vi "A170316-11-Main-large.vi"() -> ()   [LabVIEW 2020]
uses:
  System.Windows.Forms
  Database/Global1.vi
  Global_Variable/Global.vi
  <userlib>/_MGI/Menu Building/MenuTypes/MenuStrip/MGI_MenuStrip.lvclass
  <userlib>/_MGI/Menu Building/MenuItemStatusChange/MGI_MenuItemStatusChange.lvclass
  Global_Variable/A170316-11.vi
  Libraries/S7/S7.lvlib
panel:
  out "PLC":bool
  in  "模式切换":refnum<vi>
  out "管柱码":string
  out "电机自动":bool
  out "上序状态":string
  out "ECU前序显示字":string
  out "电机前序显示字":string
  out "ECU装配\n前序状态":bool
  out "上序状态":bool
  out "电机码":string
  out "电机工位管柱码":string
  out "控制器码":string
  out "ECU自动":bool
  out "电机安装数量":u32
  out "ECU结果显示":string
  out "电机结果显示":string
  in  "质量报警":bool caption="布尔"
  in  "设备缺料":bool caption="布尔"
  in  "设备故障":bool caption="布尔"
  in  "设备离线":bool caption="布尔"
  in  "设备正常":bool caption="布尔"
  in  "菜单":refnum<k24>(container)
  out "检测结果":bool
  in  "批次信息":string[][](table)
  out "提示信息":string
  out "错误":bool
  out "时间字符串":string
  out "日期字符串":string
  out "userStatus":string caption="用户状态"
  out "userName":string caption="用户名"
  out "安装支架数量":u32
  out "ECU工位管柱码":string
  out "connectionMode":string caption="联机类型"
  out "产品型号":string
  in  "更换产品":refnum<vi>
  # "调节机构装配"
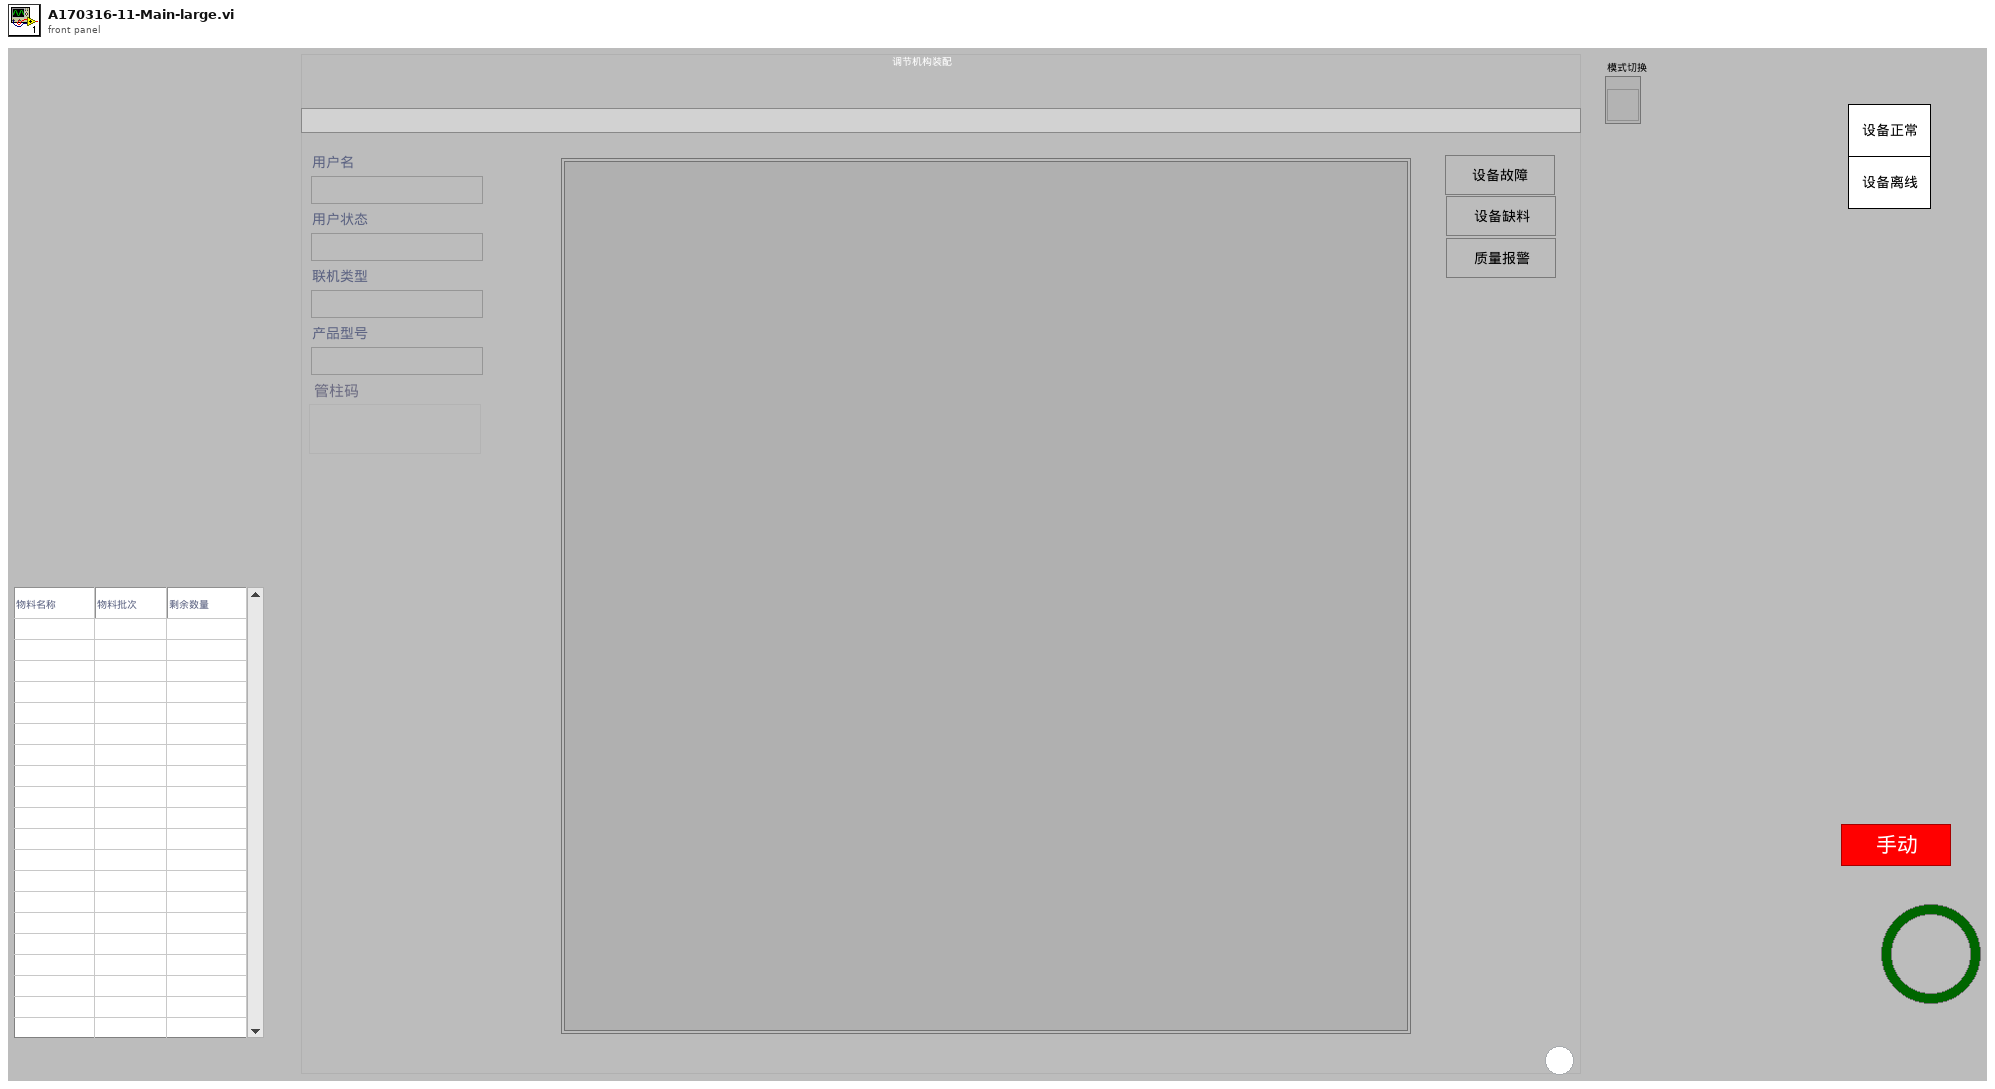
[diagram p1: front panel]
types:
  T1 = typedef "S7.lvlib/Broadcast Events--cluster.ctl" = cluster{"Module Did Init":refnum<user-event>, "Status Updated":refnum<user-event>, "Error Reported":refnum<user-event>, "Module Did Stop":refnum<user-event>, "Update Module Execution Status":refnum<user-event>}
  T2 = enum32{"Invalid", "Standard", "Closed", "Hidden", "Minimized", "Maximized"}
  T3 = enum32{"invalid app kind", "Development System", "Run Time System", "Student Edition", "Embedded LabVIEW", "Evaluation", "Custom"}
  T4 = cluster{"Core":cluster{"Current VI Reference":refnum<vi>, "Close Panel on Exit?":bool}, "Your Boolean data":bool, "Your string data":string}
  T5 = cluster{"Current VI Reference":refnum<vi>, "Close Panel on Exit?":bool}
  T6 = cluster{"用户编号":string, "用户名":string, "用户密码(密文)":string, "用户权限":string}
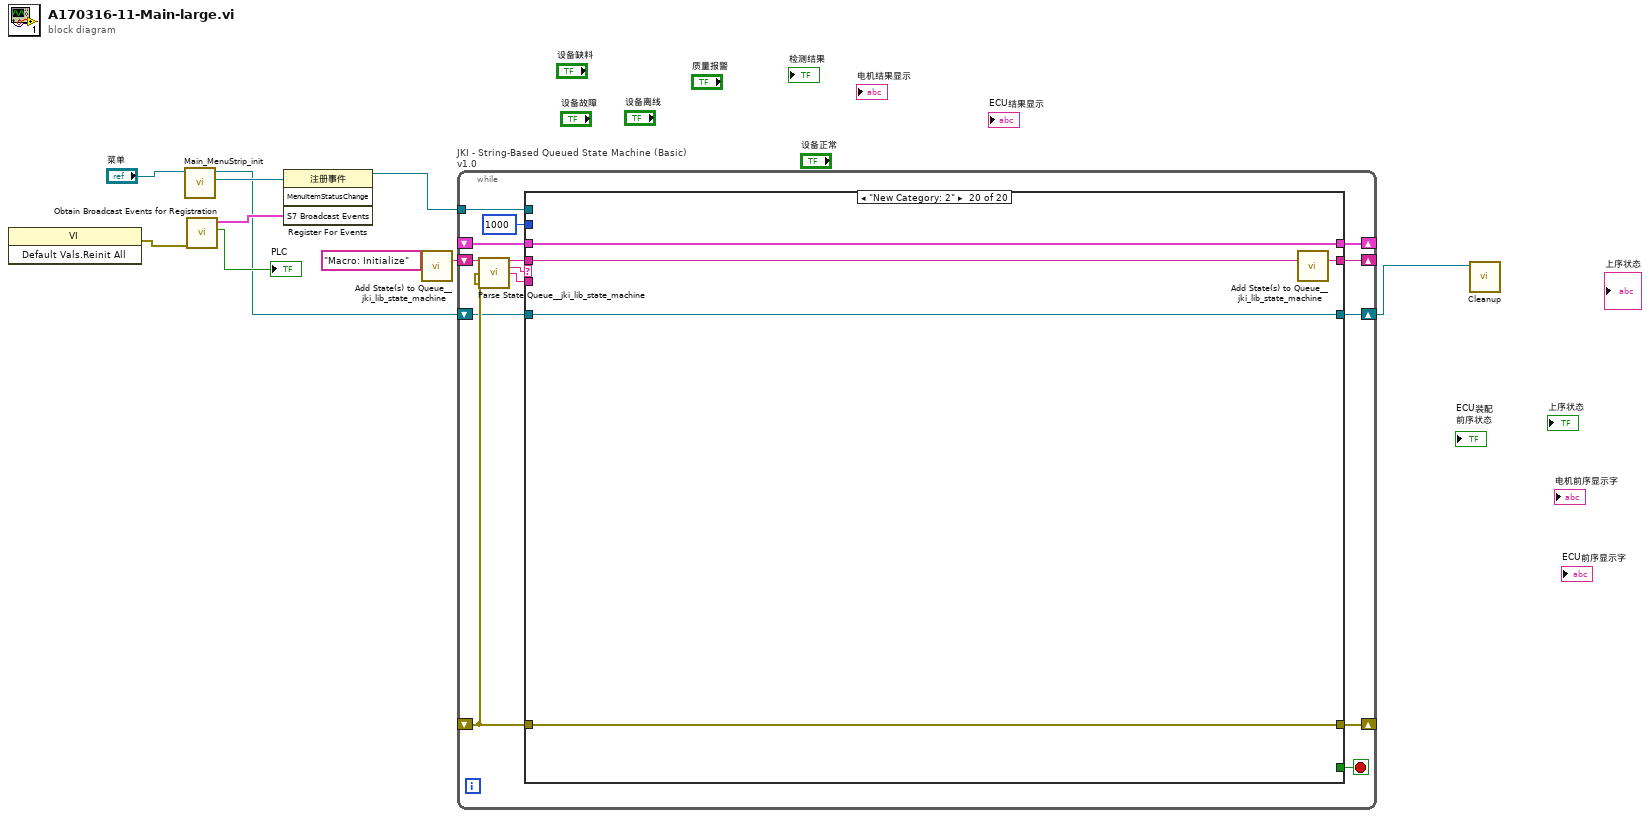
[diagram p0: block diagram]
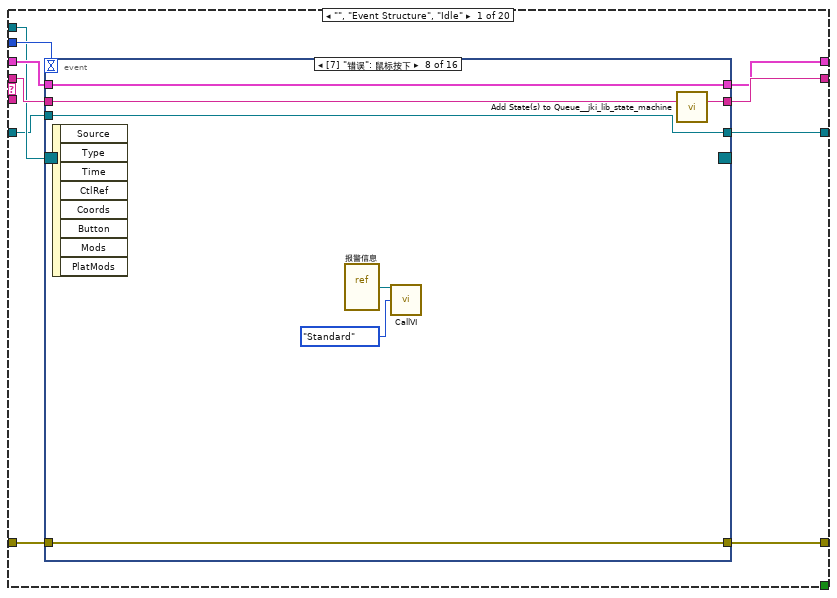
[diagram p2: hidden frame]
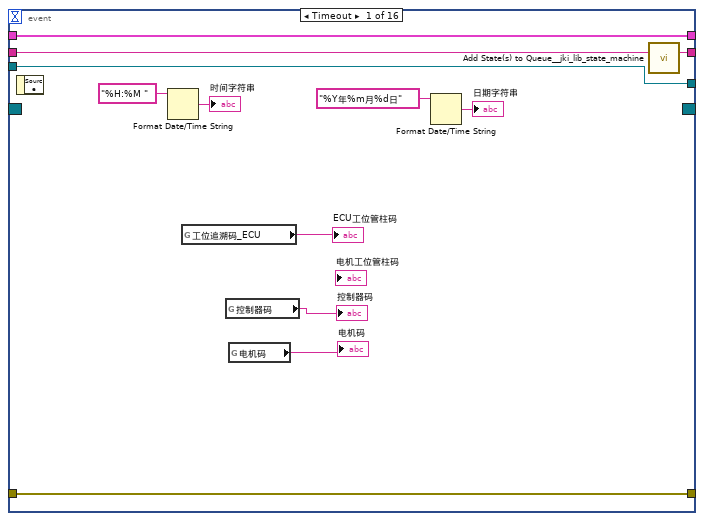
[diagram p3: hidden frame]
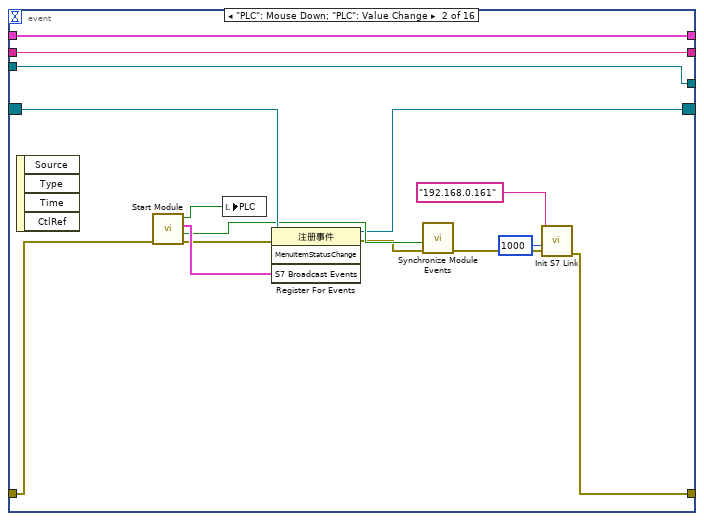
[diagram p4: hidden frame]
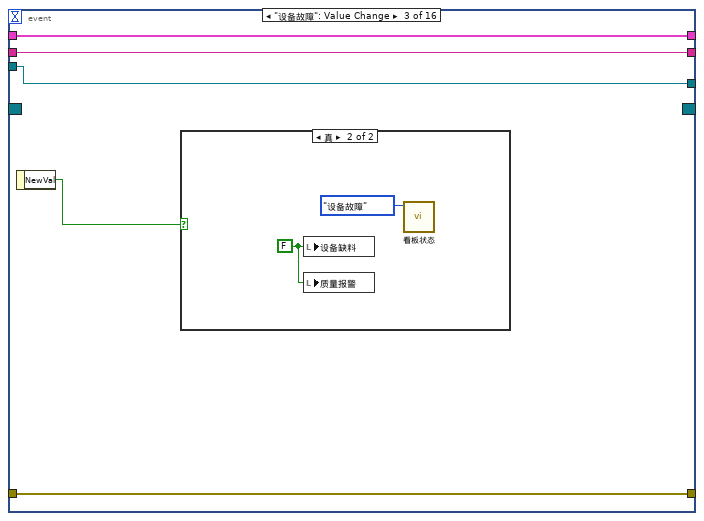
[diagram p5: hidden frame]
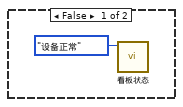
[diagram p6: hidden frame]
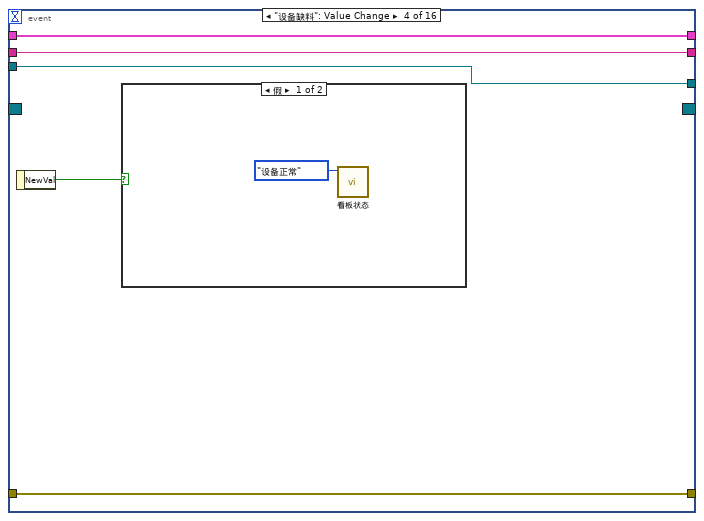
[diagram p7: hidden frame]
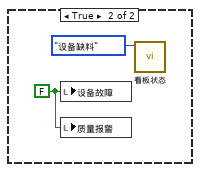
[diagram p8: hidden frame]
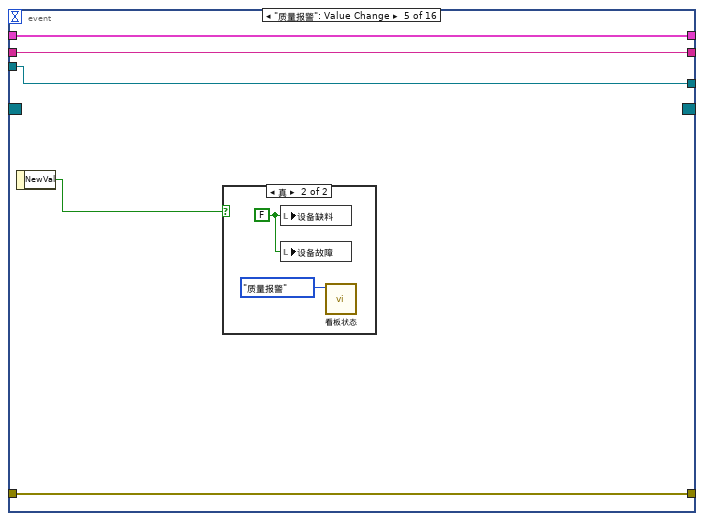
[diagram p9: hidden frame]
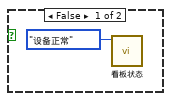
[diagram p10: hidden frame]
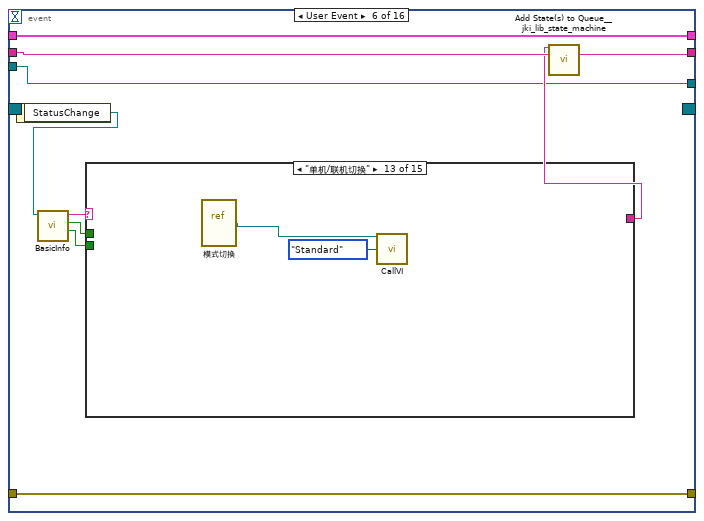
[diagram p11: hidden frame]
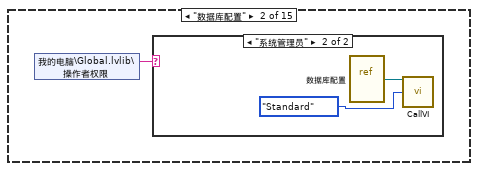
[diagram p13: hidden frame]
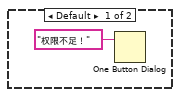
[diagram p14: hidden frame]
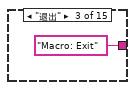
[diagram p15: hidden frame]
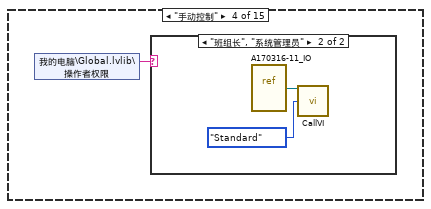
[diagram p16: hidden frame]
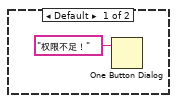
[diagram p17: hidden frame]
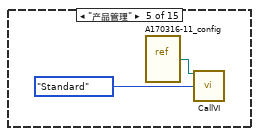
[diagram p18: hidden frame]
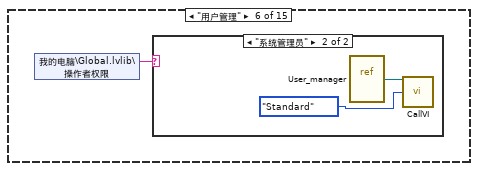
[diagram p19: hidden frame]
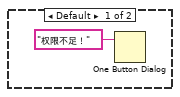
[diagram p20: hidden frame]
diagram:
  n1 = invoke class="VI" method="Default Vals.Reinit All"() -> (error out=w3:errorcluster)  [unwired: 3 in, 2 out]
  n2 = call "Main_MenuStrip_init.vi"("MenuStrip"="菜单") -> ("MenuItemStatusChange"=w6:refnum<user-event>, "Menu out"=w2:refnum<class "MGI_MenuStrip.lvclass">)  [unwired: 9 in]
  n3 = call "Obtain Broadcast Events for Registration.vi"("error in (no error)"=w3) -> ("Already running?"=→"PLC":bool, "S7 Broadcast Events"=w5:T1)  [unwired: 8 in, 1 out]
  n4 = register-events(w6, w5) -> (reference out=w7:refnum<event-registration>)  [unwired: 2 in, 1 out]
  n5 = call <vilib>:"Add State(s) to Queue__jki_lib_state_machine.vi"("State(s) in (\"\")"="Macro: Initialize") -> ("States Out"=w10:string)  [unwired: 14 in]
  n6 = while "JKI - String-Based Queued State Machine (Basic) v1.0" {
    shift-right: [w17] -> _
    shift-left: _ -> [w16]
    shift-right: [w20] -> _
    shift-left: _ -> [w14]
    shift-right: [w19] -> _
    shift-left: w10 -> [w21]
    tunnel: w7 -> [w13]
    shift-right: [w11] -> w1
    shift-left: w2 -> [w12]
    stop <- w18 stop-if-true
    n7 = call <vilib>:"Parse State Queue__jki_lib_state_machine.vi"("State Queue"=w21, "Error In (no error)"=w14) -> ("Remaining States"=w23:string, "Current State"=w24:string, "Arguments"=w22:string)  [unwired: 11 in]
    n8 = case shown="\"New Category: 2\"" w24 {
      selector: w24 -> [_ _ w268 _ _ _ _ _ _ _ _ _ _ _ _ _ _ _ _ _]
      tunnel: w23 -> [w34 w266 w272 w291 w298 w304 w309 w317 w324 w329 w342 w347 w407 w419 w446 w452 w468 w473 w478 w483]
      tunnel: w22 -> [_ _ _ _ _ _ _ _ _ _ _ _ w402 w413 _ _ _ _ _ _]
      tunnel: w16 -> [w32 w263 w270 w282 w295 w302 w306 _ w319 w326 w340 w345 w405 w415 w443 w449 w465 w470 w475 w480]
      tunnel: [w31 w264 w274 w288 errorcluster {"status"=FALSE, "code"=0, "source"=""} ("error out") w301 w307 w314 w320 w327 w339 w344 w403 w416 w444 w450 w466 w471 w476 w481] -> w20
      tunnel: w14 -> [w30 w264 w273 w288 w294 w301 w307 w314 w321 w327 w338 w344 w404 w417 w444 w450 w466 w471 w476 w481]
      tunnel: [w33 w265 w271 w290 w297 w303 w308 w316 w323 w328 w341 w346 w406 w418 w445 w451 w467 w472 w477 w482] -> w19
      tunnel: [_ _ _ _ _ TRUE _ _ _ _ _ _ _ _ _ _ _ _ _ _] -> w18
      tunnel: [w29 w263 w270 w289 w295 w302 w306 w315 w319 w326 w340 w345 w405 w415 w443 w449 w465 w470 w475 w480] -> w17
      tunnel: 1000 ("Timeout") -> [w28 _ _ _ _ _ _ _ _ _ _ _ _ _ _ _ _ _ _ _]
      tunnel: w13 -> [w27 _ _ _ _ _ _ _ _ _ _ _ _ _ _ _ _ _ _ _]
      tunnel: w12 -> [w26 w262 w267 w279 w292 w299 w305 w310 w318 w325 w330 w343 w401 w412 w442 w447 w453 w469 w474 w479]
      tunnel: [w25 w262 w267 w279 w292 w299 w305 w310 w318 w325 w330 w343 w401 w412 w442 w447 w453 w469 w474 w479] -> w11
      frame "", "Event Structure", "Idle" {
        n9 = event shown="[7] \"错误\": 鼠标按下" {
          selector: w27 -> [_ w59 _ _ _ _ _ _ _ _ _ _ _ _ _ _]
          dyn-events: [_ w50 _ _ _ _ _ _ _ _ _ _ _ _ _ _] -> _
          timeout: w28 -> [_ _ _ _ _ _ _ _ _ _ _ _ _ _ _ _]
          tunnel: w34 -> [w46 w48 w65 w73 w81 w90 w143 w194 w201 w225 w229 w234 w239 w246 w255 w258]
          tunnel: [w45 w48 w65 w73 w81 w89 w141 w195 w201 w225 w229 w234 w239 w244 w254 w259] -> w33
          tunnel: w32 -> [w43 w49 w66 w74 w82 w91 w142 w196 w202 w226 w228 w235 w240 w245 w252 w261]
          tunnel: [w44 w51 w64 w72 w80 w87 w144 w193 w200 w224 w227 w232 w237 w242 w253 w260] -> w31
          tunnel: w30 -> [w44 w61 w64 w72 w80 w87 w144 w193 w200 w224 w227 w232 w237 w242 w253 w260]
          tunnel: [w43 w49 w66 w74 w82 w91 w142 w196 w202 w226 w228 w235 w240 w245 w252 w261] -> w29
          tunnel: w26 -> [w35 w47 w62 w70 w78 w86 w140 w190 w197 w223 w230 w233 w238 w243 _ _]
          tunnel: [w35 w47 w62 w70 w78 w86 w140 w190 w197 w223 w230 w233 w238 w243 _ _] -> w25
          event Timeout {
            n10 = event-data() -> ()  [unwired: 1 in, 1 out]
            n11 = Format Date/Time String(time format string (%c)="%H:%M ") -> (date/time string=→"时间字符串":string)  [unwired: 2 in]
            n12 = global read "Global1.vi" "工位追溯码_ECU"() -> (→"ECU工位管柱码":string)
            n13 = global read "Global1.vi" "控制器码"() -> (→"控制器码":string)
            n14 = global read "Global1.vi" "电机码"() -> (→"电机码":string)
            n15 = Format Date/Time String(time format string (%c)="%Y年%m月%d日") -> (date/time string=→"日期字符串":string)  [unwired: 2 in]
            n16 = call <vilib>:"Add State(s) to Queue__jki_lib_state_machine.vi"("State(s) in (\"\")"=w46) -> ("States Out"=w45:string)  [unwired: 14 in]
          }
          event "PLC": Mouse Down; "PLC": Value Change {
            n17 = event-data() -> ()  [unwired: 1 in, 4 out]
            n18 = call "Start Module.vi"("error in (no error)"=w61) -> ("error out"=w57:errorcluster, "Wait for Event Sync?"=w56:bool, "S7 Broadcast Events"=w58:T1, "Module Was Already Running?"=w60:bool)  [unwired: 7 in]
            n19 = local write "PLC"(w60) -> ()
            n20 = register-events(reference=w59, error in=w57, w58) -> (reference out=w50:refnum<event-registration>, error out=w55:errorcluster)  [unwired: 1 in]
            n21 = call "Synchronize Module Events.vi"("error in (no error)"=w55, "Wait for Event Sync?"=w56) -> ("error out"=w54:errorcluster)  [unwired: 9 in]
            n22 = call "Init S7 Link.vi"("error in (no error)"=w54, "超时"=1000, "IP"="192.168.0.161") -> ("error out"=w51:errorcluster)  [unwired: 8 in]
          }
          event "设备故障": Value Change {
            n23 = event-data() -> ("NewVal"=w63:bool)  [unwired: 1 in]
            n24 = case shown="真" w63 {
              frame False {
                n25 = call "看板状态.vi"("设备状态"=enum16{"设备离线", "设备正常", "设备缺料", "设备故障", "质量报警"}."设备正常") -> ()  [unwired: 10 in, 1 out]
              }
              frame True {
                w68 = FALSE ("质量报警")
                n26 = local write "设备缺料"(w68) -> ()
                n27 = local write "质量报警"(w68) -> ()
                n28 = call "看板状态.vi"("设备状态"=enum16{"设备离线", "设备正常", "设备缺料", "设备故障", "质量报警"}."设备故障") -> ()  [unwired: 10 in, 1 out]
              }
            }
          }
          event "设备缺料": Value Change {
            n29 = event-data() -> ("NewVal"=w71:bool)  [unwired: 1 in]
            n30 = case shown="假" w71 {
              frame False {
                n31 = call "看板状态.vi"("设备状态"=enum16{"设备离线", "设备正常", "设备缺料", "设备故障", "质量报警"}."设备正常") -> ()  [unwired: 10 in, 1 out]
              }
              frame True {
                w76 = FALSE ("质量报警")
                n32 = local write "设备故障"(w76) -> ()
                n33 = local write "质量报警"(w76) -> ()
                n34 = call "看板状态.vi"("设备状态"=enum16{"设备离线", "设备正常", "设备缺料", "设备故障", "质量报警"}."设备缺料") -> ()  [unwired: 10 in, 1 out]
              }
            }
          }
          event "质量报警": Value Change {
            n35 = event-data() -> ("NewVal"=w79:bool)  [unwired: 1 in]
            n36 = case shown="真" w79 {
              frame False {
                n37 = call "看板状态.vi"("设备状态"=enum16{"设备离线", "设备正常", "设备缺料", "设备故障", "质量报警"}."设备正常") -> ()  [unwired: 10 in, 1 out]
              }
              frame True {
                w84 = FALSE ("质量报警")
                n38 = local write "设备缺料"(w84) -> ()
                n39 = local write "设备故障"(w84) -> ()
                n40 = call "看板状态.vi"("设备状态"=enum16{"设备离线", "设备正常", "设备缺料", "设备故障", "质量报警"}."质量报警") -> ()  [unwired: 10 in, 1 out]
              }
            }
          }
          event User Event {
            n41 = event-data() -> ("StatusChange"=w92:refnum<class "MGI_MenuItemStatusChange.lvclass">)  [unwired: 1 in]
            n42 = call <userlib>:"BasicInfo.vi"("MGI_MenuItemStatusChange in"=w92) -> ("Enabled?"=w95:bool, "Checked?"=w94:bool, "Tag"=w93:string)  [unwired: 7 in, 1 out]
            n43 = case shown="\"单机/联机切换\"" w93 {
              tunnel: w94 -> [_ _ _ _ _ _ _ _ _ _ _ _ _ _ _]
              tunnel: w95 -> [_ _ _ _ _ _ _ _ _ _ _ _ _ _ _]
              tunnel: [_ _ "Macro: Exit" _ _ _ _ _ _ _ _ _ _ _ _] -> w88
              frame Default {
              }
              frame "数据库配置" {
                n44 = shared-variable "我的电脑\\Global.lvlib\\操作者权限"() -> (w96:string)  [unwired: 1 in, 1 out]
                n45 = case shown="\"系统管理员\"" w96 {
                  frame Default {
                    n46 = One Button Dialog(message="权限不足！" ("消息")) -> ()  [unwired: 1 in, 1 out]
                  }
                  frame "系统管理员" {
                    n47 = vi-ref "数据库配置.vi"() -> (w99:refnum<vi>)
                    n48 = call "CallVI.vi"("VI引用"=w99, "状态"=T2."Standard") -> ()  [unwired: 11 in, 3 out]
                  }
                }
              }
              frame "退出" {
              }
              frame "手动控制" {
                n49 = shared-variable "我的电脑\\Global.lvlib\\操作者权限"() -> (w101:string)  [unwired: 1 in, 1 out]
                n50 = case shown="\"班组长\", \"系统管理员\"" w101 {
                  frame Default {
                    n51 = One Button Dialog(message="权限不足！" ("消息")) -> ()  [unwired: 1 in, 1 out]
                  }
                  frame "班组长", "系统管理员" {
                    n52 = vi-ref "A170316-11_IO.vi"() -> (w104:refnum<vi>)
                    n53 = call "CallVI.vi"("VI引用"=w104, "状态"=T2."Standard") -> ()  [unwired: 11 in, 3 out]
                  }
                }
              }
              frame "产品管理" {
                n54 = vi-ref "A170316-11_config.vi"() -> (w106:refnum<vi>)
                n55 = call "CallVI.vi"("VI引用"=w106, "状态"=T2."Standard") -> ()  [unwired: 11 in, 3 out]
              }
              frame "用户管理" {
                n56 = shared-variable "我的电脑\\Global.lvlib\\操作者权限"() -> (w107:string)  [unwired: 1 in, 1 out]
                n57 = case shown="\"系统管理员\"" w107 {
                  frame Default {
                    n58 = One Button Dialog(message="权限不足！" ("消息")) -> ()  [unwired: 1 in, 1 out]
                  }
                  frame "系统管理员" {
                    n59 = vi-ref "User_manager.vi"() -> (w110:refnum<vi>)
                    n60 = call "CallVI.vi"("VI引用"=w110, "状态"=T2."Standard") -> ()  [unwired: 11 in, 3 out]
                  }
                }
              }
              frame "编码规则" {
                n61 = shared-variable "我的电脑\\Global.lvlib\\操作者权限"() -> (w111:string)  [unwired: 1 in, 1 out]
                n62 = case shown="\"班组长\", \"工艺管理员\", \"系统管理员\"" w111 {
                  frame Default {
                    n63 = One Button Dialog(message="权限不足！" ("消息")) -> ()  [unwired: 1 in, 1 out]
                  }
                  frame "班组长", "工艺管理员", "系统管理员" {
                    n64 = vi-ref "编码规则设置.vi"() -> (w114:refnum<vi>)
                    n65 = call "CallVI.vi"("VI引用"=w114, "状态"=T2."Standard") -> ()  [unwired: 11 in, 3 out]
                  }
                }
              }
              frame "易损件管理" {
                n66 = vi-ref "易损件管理.vi"() -> (w116:refnum<vi>)
                n67 = call "CallVI.vi"("VI引用"=w116, "状态"=T2."Standard") -> ()  [unwired: 11 in, 3 out]
              }
              frame "物料批次管理" {
                n68 = vi-ref "批次管理.vi"() -> (w118:refnum<vi>)
                n69 = call "CallVI.vi"("VI引用"=w118, "状态"=T2."Standard") -> ()  [unwired: 11 in, 3 out]
              }
              frame "设备管理" {
                n70 = vi-ref "注册设备.vi"() -> (w120:refnum<vi>)
                n71 = call "CallVI.vi"("VI引用"=w120, "状态"=T2."Standard") -> ()  [unwired: 11 in, 3 out]
              }
              frame "报表" {
                n72 = call "文件对话框2"("start path"=path "D:/report", "prompt"="打开报表", "pattern (all files)"="*.doc;*.docx", "pattern label"="Word 文档") -> ("selected path"=w121:path, "error out"=w122:errorcluster)  [unwired: 8 in, 2 out]
                n73 = case shown="无错误" w122 {
                  selector: w122 -> [w128 w130]
                  tunnel: w121 -> [w129 _]
                  frame No Error {
                    w127 = 1 items=["Normal", "Maximize", "Minimize"] ("cpubbs_WindowState")
                    n74 = call "Open_Word.vi"("File Path"=w129, "cpubbs_WindowState"=w127, "错误输入（无错误）"=w128) -> ()  [unwired: 12 in, 1 out]
                  }
                  frame Error {
                    n75 = call <vilib>:"Clear Errors.vi"("error in (no error)"=w130) -> ()  [unwired: 5 in, 2 out]
                  }
                }
              }
              frame "报警信息" {
                n76 = vi-ref "报警信息.vi"() -> (w132:refnum<vi>)
                n77 = call "CallVI.vi"("VI引用"=w132, "状态"=T2."Standard") -> ()  [unwired: 11 in, 3 out]
              }
              frame "单机/联机切换" {
                n78 = vi-ref "模式切换.vi"() -> (w133:refnum<vi>)
                n79 = call "CallVI.vi"("VI引用"=w133, "状态"=T2."Standard") -> ()  [unwired: 11 in, 3 out]
              }
              frame "关于" {
                n80 = vi-ref "About.vi"() -> (w136:refnum<vi>)
                n81 = call "CallVI.vi"("VI引用"=w136, "状态"=T2."Standard") -> ()  [unwired: 11 in, 3 out]
              }
              frame "操作演示" {
                n82 = call <vilib>:"Application Directory.vi"() -> ("Application Directory"=w139:path)
                n83 = Build Path(base path=w139, name or relative path="操作演示" ("名称或相对路径")) -> (appended path=w138:path)
                n84 = call "自动播放ppt.vi"("路径"=w138) -> ()  [unwired: 10 in, 1 out]
              }
            }
            n85 = call <vilib>:"Add State(s) to Queue__jki_lib_state_machine.vi"("State(s) in Front (\"\")"=w88, "State(s) in (\"\")"=w90) -> ("States Out"=w89:string)  [unwired: 13 in]
          }
          event Menu Selection (User) {
            n86 = event-data() -> ("ItemTag"=w145:string)  [unwired: 1 in, 6 out]
            n87 = case shown="\"易损件管理\"" w145 {
              frame "假", Default {
              }
              frame "数据库配置" {
                n88 = shared-variable "我的电脑\\Global.lvlib\\操作者权限"() -> (w146:string)  [unwired: 1 in, 1 out]
                n89 = case shown="\"系统管理员\"" w146 {
                  frame Default {
                    n90 = One Button Dialog(message="权限不足！" ("消息")) -> ()  [unwired: 1 in, 1 out]
                  }
                  frame "系统管理员" {
                    n91 = vi-ref "数据库配置.vi"() -> (w149:refnum<vi>)
                    n92 = call "CallVI.vi"("VI引用"=w149, "状态"=T2."Standard") -> ()  [unwired: 11 in, 3 out]
                  }
                }
              }
              frame "退出" {
                n93 = Quit LabVIEW() -> ()  [unwired: 1 in]
              }
              frame "手动控制" {
                n94 = shared-variable "我的电脑\\Global.lvlib\\操作者权限"() -> (w150:string)  [unwired: 1 in, 1 out]
                n95 = case shown="\"班组长\", \"系统管理员\"" w150 {
                  frame Default {
                    n96 = One Button Dialog(message="权限不足！" ("消息")) -> ()  [unwired: 1 in, 1 out]
                  }
                  frame "班组长", "系统管理员" {
                    n97 = vi-ref "A170316-11_IO.vi"() -> (w153:refnum<vi>)
                    n98 = call "CallVI.vi"("VI引用"=w153, "状态"=T2."Standard") -> ()  [unwired: 11 in, 3 out]
                  }
                }
              }
              frame "半自动控制" {
                n99 = disable-structure shown="启用" {
                  frame Disabled {
                    n100 = shared-variable "我的电脑\\Global.lvlib\\操作者权限"() -> (w154:string)  [unwired: 1 in, 1 out]
                    n101 = case shown="\"班组长\", \"系统管理员\"" w154 {
                      frame Default {
                        n102 = One Button Dialog(message="权限不足！" ("消息")) -> ()  [unwired: 1 in, 1 out]
                      }
                      frame "班组长", "系统管理员" {
                        n103 = call "CallVI.vi"("VI引用"=refnum<vi> refnum, "状态"=T2."Maximized") -> ()  [unwired: 11 in, 3 out]
                      }
                    }
                  }
                  frame Enabled {
                    n104 = One Button Dialog(message="当前设备不具备半自动功能！" ("消息")) -> ()  [unwired: 1 in, 1 out]
                  }
                }
              }
              frame "产品管理" {
                n105 = vi-ref "A170316-11_config.vi"() -> (w160:refnum<vi>)
                n106 = call "CallVI.vi"("VI引用"=w160, "状态"=T2."Standard") -> ()  [unwired: 11 in, 3 out]
              }
              frame "系统配置" {
              }
              frame "用户管理" {
                n107 = shared-variable "我的电脑\\Global.lvlib\\操作者权限"() -> (w161:string)  [unwired: 1 in, 1 out]
                n108 = case shown="\"系统管理员\"" w161 {
                  frame Default {
                    n109 = One Button Dialog(message="权限不足！" ("消息")) -> ()  [unwired: 1 in, 1 out]
                  }
                  frame "系统管理员" {
                    n110 = vi-ref "User_manager.vi"() -> (w164:refnum<vi>)
                    n111 = call "CallVI.vi"("VI引用"=w164, "状态"=T2."Standard") -> ()  [unwired: 11 in, 3 out]
                  }
                }
              }
              frame "编码规则" {
                n112 = shared-variable "我的电脑\\Global.lvlib\\操作者权限"() -> (w165:string)  [unwired: 1 in, 1 out]
                n113 = case shown="\"班组长\", \"工艺管理员\", \"系统管理员\"" w165 {
                  frame Default {
                    n114 = One Button Dialog(message="权限不足！" ("消息")) -> ()  [unwired: 1 in, 1 out]
                  }
                  frame "班组长", "工艺管理员", "系统管理员" {
                    n115 = vi-ref "编码规则设置.vi"() -> (w168:refnum<vi>)
                    n116 = call "CallVI.vi"("VI引用"=w168, "状态"=T2."Standard") -> ()  [unwired: 11 in, 3 out]
                  }
                }
              }
              frame "易损件管理" {
                n117 = vi-ref "易损件管理.vi"() -> (w170:refnum<vi>)
                n118 = call "CallVI.vi"("VI引用"=w170, "状态"=T2."Standard") -> ()  [unwired: 11 in, 3 out]
              }
              frame "物料批次管理" {
                n119 = vi-ref "批次管理.vi"() -> (w172:refnum<vi>)
                n120 = call "CallVI.vi"("VI引用"=w172, "状态"=T2."Standard") -> ()  [unwired: 11 in, 3 out]
              }
              frame "打开报表" {
                n121 = call "文件对话框"("start path"=path "D:/report", "prompt"="打开报表", "pattern (all files)"="*.doc;*.docx", "pattern label"="Word 文档") -> ("selected path"=w173:path, "error out"=w174:errorcluster)  [unwired: 8 in, 2 out]
                n122 = case shown="无错误" w174 {
                  selector: w174 -> [w180 w182]
                  tunnel: w173 -> [w181 _]
                  frame No Error {
                    w179 = 1 items=["Normal", "Maximize", "Minimize"] ("cpubbs_WindowState")
                    n123 = call "Open_Word.vi"("File Path"=w181, "cpubbs_WindowState"=w179, "错误输入（无错误）"=w180) -> ()  [unwired: 12 in, 1 out]
                  }
                  frame Error {
                    n124 = call <vilib>:"Clear Errors.vi"("error in (no error)"=w182) -> ()  [unwired: 5 in, 2 out]
                  }
                }
              }
              frame "报警信息" {
                n125 = vi-ref "报警信息.vi"() -> (w184:refnum<vi>)
                n126 = call "CallVI.vi"("VI引用"=w184, "状态"=T2."Standard") -> ()  [unwired: 11 in, 3 out]
              }
              frame "关于" {
                n127 = vi-ref "About.vi"() -> (w186:refnum<vi>)
                n128 = call "CallVI.vi"("VI引用"=w186, "状态"=T2."Standard") -> ()  [unwired: 11 in, 3 out]
              }
              frame "操作演示" {
                n129 = call <vilib>:"Application Directory.vi"() -> ("Application Directory"=w189:path)
                n130 = Build Path(base path=w189, name or relative path="操作演示" ("名称或相对路径")) -> (appended path=w188:path)
                n131 = call "自动播放ppt.vi"("路径"=w188) -> ()  [unwired: 10 in, 1 out]
              }
            }
            n132 = call <vilib>:"Add State(s) to Queue__jki_lib_state_machine.vi"("State(s) in (\"\")"=w143) -> ("States Out"=w141:string)  [unwired: 14 in]
          }
          event "错误": Mouse Down {
            n133 = event-data() -> ()  [unwired: 1 in, 8 out]
            n134 = vi-ref "报警信息.vi"() -> (w192:refnum<vi>)
            n135 = call "CallVI.vi"("VI引用"=w192, "状态"=T2."Standard") -> ()  [unwired: 11 in, 3 out]
            n136 = call <vilib>:"Add State(s) to Queue__jki_lib_state_machine.vi"("State(s) in (\"\")"=w194) -> ("States Out"=w195:string)  [unwired: 14 in]
          }
          event "电机自动": Mouse Down {
            n137 = event-data() -> ("CtlRef"=w199:refnum<vi>)  [unwired: 1 in, 7 out]
            n138 = property class="Bool (严格)"(reference=w199) -> ("Value"=w198:bool)  [unwired: 1 in, 2 out]
            n139 = disable-structure shown="禁用" {
              disable-tunnel: w198 -> [w203 _]
              frame Disabled {
                n140 = case shown="真" w203 {
                  frame False {
                    n141 = shared-variable "我的电脑\\240调节机构装配.lvlib\\设备状态"() -> (w204:u16)  [unwired: 1 in, 1 out]
                    n142 = case shown="5" w204 {
                      frame 0, Default {
                        n143 = call "浮动通知.vi"("通知内容"="请复位！") -> ()  [unwired: 11 in]
                      }
                      frame 5 {
                      }
                    }
                  }
                  frame True {
                    n144 = global read "A170316-11.vi" "手柄安装LED"() -> (w207:refnum<vi>[])
                    n145 = global read "A170316-11.vi" "安装支架LED"() -> (w208:refnum<vi>[])
                    n146 = global read "A170316-11.vi" "控制器支架LED"() -> (w206:refnum<vi>[])
                    n147 = Two Button Dialog(message="自动程序运行中，\n是否切换为手动？" ("消息")) -> (T button?=w209:bool)  [unwired: 2 in]
                    n148 = case shown="真" w209 {
                      tunnel: w208 -> [_ w216]
                      tunnel: w207 -> [_ w215]
                      tunnel: w206 -> [_ w214]
                      frame False {
                      }
                      frame True {
                        n149 = for {
                          tunnel: w216 -> [w221] mode=indexing
                          n150 = call "Colour.vi"("result"="", "colourRef"=w221) -> ()  [unwired: 9 in, 1 out]
                        }
                        n151 = vi-ref "A170316-11_Auto.vi"() -> (w213:refnum<vi>)
                        n152 = for {
                          tunnel: w214 -> [w217] mode=indexing
                          n153 = call "Colour.vi"("result"="", "colourRef"=w217) -> ()  [unwired: 9 in, 1 out]
                        }
                        n154 = invoke class="VI" method="Ctrl Val.Set"(reference=w213, "Control Name"="STEP3" ("控件名"), "Value"="手动" ("控件名")) -> ()  [unwired: 2 in, 5 out]
                        n155 = for {
                          tunnel: w215 -> [w219] mode=indexing
                          n156 = call "Colour.vi"("result"="", "colourRef"=w219) -> ()  [unwired: 9 in, 1 out]
                        }
                      }
                    }
                  }
                }
              }
              frame Enabled {
              }
            }
          }
          event "ECU自动": Mouse Down {
            n157 = event-data() -> ()  [unwired: 1 in, 8 out]
          }
          event User Event {
            n158 = event-data() -> ("Init?"=w231:bool)  [unwired: 1 in, 5 out]
            n159 = local write "PLC"(w231) -> ()
          }
          event User Event {
            n160 = event-data() -> ("Running?"=w236:bool)  [unwired: 1 in, 4 out]
            n161 = local write "PLC"(w236) -> ()
          }
          event User Event {
            n162 = event-data() -> ()  [unwired: 1 in, 7 out]
            n163 = local write "PLC"(FALSE ("PLC")) -> ()
          }
          event User Event {
            n164 = event-data() -> ()  [unwired: 1 in, 1 out]
            n165 = call <vilib>:"Add State(s) to Queue__JKI_lib_State_Machine.vi"("State(s) in Front (\"\")"="S7: Initialize\nIdle" ("State(s) in Front (\"\")"), "State(s) in (\"\")"=w246) -> ("States Out"=w244:string)  [unwired: 13 in]
          }
          event Panel Close? {
            n166 = event-data() -> ()  [unwired: 1 in, 1 out]
            n167 = control-ref of="本VI"() -> (w248:refnum<vi>)
            n168 = invoke class="VI" method="FP.Close"(reference=w248) -> ()  [unwired: 2 in, 3 out]
            n169 = global write "Global.vi" "程序关闭"(TRUE ("程序关闭")) -> ()
            n170 = event-data("Discard?"=TRUE) -> ()  [unwired: 1 in, 1 out]
            n171 = call <vilib>:"Add State(s) to Queue__jki_lib_state_machine.vi"("State(s) in Front (\"\")"="Macro: Exit", "State(s) in (\"\")"=w255) -> ("States Out"=w254:string)  [unwired: 13 in]
          }
          event "更换产品": Value Change {
            n172 = event-data() -> ("NewVal"=w257:refnum<vi>)  [unwired: 1 in, 5 out]
            n173 = control-ref of="子面板"() -> (w256:refnum<vi>)
            n174 = call "Call_SubPanal.vi"("VI引用句柄"=w257, "SubPnl引用句柄"=w256) -> ()  [unwired: 9 in, 1 out]
            n175 = call <vilib>:"Add State(s) to Queue__jki_lib_state_machine.vi"("State(s) in (\"\")"=w258) -> ("States Out"=w259:string)  [unwired: 14 in]
          }
        }
      }
      frame "---------- Core ----------" {
        n176 = call <vilib>:"Add State(s) to Queue__jki_lib_state_machine.vi"("State(s) in (\"\")"=w266) -> ("States Out"=w265:string)  [unwired: 14 in]
      }
      frame Default {
        w277 = 42 items=["No error", "Argument error", "Memory is full", "Out of zone", "End of file", "File already open", "Generic file I/O error", "File not found", "File permission error", "Disk is full", "Duplicate path", "Too many files open", "System feature not enabled", "Resource file not found", "Cannot add resource", "Resource not found", "Image not found", "Image memory error", "Pen does not exist", "Config type invalid", "Config token not found", "Config parse error", "Config memory error", "Bad external code format", "Bad external code offset", "External code not present", "Null window", "Destroy window error", "Null menu", "Print aborted", "Bad print record", "Print driver error", "Windows error during printing", "Memory error during printing", "Print dialog error", "Generic print error", "Invalid device refnum", "Device not found", "Device parameter error", "Device unit error", "Cannot open device", "Device call aborted", "Generic error", "Cancelled by user", "Object ID too low", "Object ID too high", "Object not in heap", "Unknown heap", "Unknown object (invalid DefProc)", "Unknown object (DefProc not in table)", "Message out of range", "Invalid (null) method", "Unknown message", "Manager call not supported", "Bad address", "Network operation in progress", "Network operation timed out", "Connection is busy", "Network attribute not supported", "Network error", "Address in use", "System out of memory", "Connection aborted", "Connection refused", "Not connected", "Already connected", "Connection closed", "Initialization error (interapplication manager)", "Bad occurrence", "Wait on unbound occurrence handler", "Occurrence queue overflow", "Datalog type conflict", "Unused", "Unrecognized type (interapplication manager)", "Memory corrupt", "Failed to make temporary DLL", "Old CIN version", "Drag socket not found", "Failed to load drop-object", "Failed to register OLE object", "Failed to release OLE object", "Format specifier type mismatch", "Unknown format specifier", "Too few format specifiers", "Too many format specifiers", "Scan failed", "Newer CIN version", "Error converting to variant", "Runtime menu error", "Password tampered", "Variant attribute not found", "Incompatible variant data type", "Event data is not available", "Event Store is not present", "Occurrence is not found", "Event Queue is not created", "Event info is not available", "Refnum passed is NULL", "Error retrieving Class GUID", "Error retrieving CoClass GUID", "Error retrieving TypeLib GUID.", "Bad built application magic bytes.", "Specific driver is different from the specific driver associated with the Logical Name.", "There is no session opened to the class driver.", "Max Error", "MAX - Error with config objects", "MAX - Error loading configuration", "MAX - Group not supported"]
        # "Current State"
        n177 = Format Into String(format string="Software Exception: Unhandled State \"%s\"." ("message"), error in=w273, w268) -> (resulting string=w276:string, error out=w275:errorcluster)  [unwired: 1 in]
        n178 = call <vilib>:"Error Cluster From Error Code.vi"("show call chain? (False)"=TRUE, "error in (no error)"=w275, "error message (\"\")"=w276, "error code (0)"=w277) -> ("error out"=w274:errorcluster)  [unwired: 5 in]
        n179 = call <vilib>:"Add State(s) to Queue__jki_lib_state_machine.vi"("State(s) in (\"\")"=w272) -> ("States Out"=w271:string)  [unwired: 14 in]
      }
      frame "Initialize Core Data" {
        # "originally closed?"
        # "exe?"
        n180 = property class="VI"() -> ("Front Panel.Open"=w287:bool)  [unwired: 2 in, 2 out]
        n181 = property class="App"() -> ("App.Kind"=w286:T3)  [unwired: 2 in, 2 out]
        n182 = control-ref of="Current VI Reference"() -> (w280:refnum<vi>)
        n183 = Not(x=w287) -> (.not. x?=w284:bool)
        n184 = Equal?(x=w286, y=T3."Run Time System" ("Application:Kind")) -> (x = y?=w283:bool)
        n185 = Or(x=w284, y=w283) -> (x .or. y?=w281:bool)
        n186 = Bundle By Name(cluster=w282, "Core.Current VI Reference"=w280, "Core.Close Panel on Exit?"=w281) -> (w289:T4)
        n187 = call <vilib>:"Add State(s) to Queue__jki_lib_state_machine.vi"("State(s) in (\"\")"=w291) -> ("States Out"=w290:string)  [unwired: 14 in]
      }
      frame "Error Handler" {
        n188 = call <vilib>:"General Error Handler.vi"("error in (no error)"=w294) -> ()  [unwired: 10 in, 5 out]
        n189 = call <vilib>:"Add State(s) to Queue__jki_lib_state_machine.vi"("State(s) in Front (\"\")"="/* Post Error States", "State(s) in (\"\")"=w298) -> ("States Out"=w297:string)  [unwired: 13 in]
      }
      frame "Exit" {
        n190 = call <vilib>:"Add State(s) to Queue__jki_lib_state_machine.vi"("State(s) in (\"\")"=w304) -> ("States Out"=w303:string)  [unwired: 14 in]
      }
      frame "---------- Data ----------" {
        n191 = call <vilib>:"Add State(s) to Queue__jki_lib_state_machine.vi"("State(s) in (\"\")"=w309) -> ("States Out"=w308:string)  [unwired: 14 in]
      }
      frame "Data: Initialize" {
        w311 = T5 {"Current VI Reference"=refnum, "Close Panel on Exit?"=FALSE}  # Core
        w313 = TRUE  # Your Boolean data
        w312 = ""  # Your string data
        n192 = Bundle("Core"=w311, "Your Boolean data"=w313, "Your string data"=w312) -> (w315:T4)  [unwired: 1 in]
        n193 = call <vilib>:"Add State(s) to Queue__jki_lib_state_machine.vi"("State(s) in (\"\")"=w317) -> ("States Out"=w316:string)  [unwired: 14 in]
      }
      frame "Data: Cleanup" {
        n194 = Unbundle By Name(w319) -> ("Core.Current VI Reference"=w322:refnum<vi>)
        n195 = Close Reference(reference=w322, error in (no error)=w321) -> (error out=w320:errorcluster)
        n196 = call <vilib>:"Add State(s) to Queue__jki_lib_state_machine.vi"("State(s) in (\"\")"=w324) -> ("States Out"=w323:string)  [unwired: 14 in]
      }
      frame "---------- UI ----------" {
        # "Do not put any code in this frame.\n(It is a separator no-op. You can make a copy of this frame to create a new UI frame)"
        n197 = call <vilib>:"Add State(s) to Queue__jki_lib_state_machine.vi"("State(s) in (\"\")"=w329) -> ("States Out"=w328:string)  [unwired: 14 in]
      }
      frame "UI: Initialize" {
        n198 = vi-ref "A170316-11_Auto.vi"() -> (w331:refnum<vi>)
        n199 = invoke on="子面板" class="SubPnl" method="Insert VI"(error in=w338, "VI Ref"=w331) -> (error out=w332:errorcluster)  [unwired: 2 in, 3 out]
        n200 = invoke class="VI" method="Run VI"(reference=w331, error in=w332, "Wait until done"=FALSE ("结束前等待"), "Auto Dispose Ref"=TRUE ("自动销毁引用")) -> (error out=w335:errorcluster)  [unwired: 1 in, 4 out]
        n201 = call "窗口自动调整.vi-.vi"("error in (no error)"=w335, "max？"=TRUE, "border spacing (2 px)"=0) -> ("error out"=w339:errorcluster)  [unwired: 3 in, 1 out]
        n202 = call <vilib>:"Add State(s) to Queue__jki_lib_state_machine.vi"("State(s) in (\"\")"=w342) -> ("States Out"=w341:string)  [unwired: 14 in]
      }
      frame "UI: Init" {
        n203 = stacked-sequence {
          frame #0 {
            w359 = u32 0 ("合格数量")
            w350 = "" ("输出轴码")
            n204 = control-ref of="管柱码"() -> (w349:refnum<vi>)
            n205 = global write "Global.vi" "管柱码"(w349) -> ()
            n206 = global read "Global1.vi" "联机模式"() -> (w348:enum16{"单机", "追溯"})
            n207 = global read "Global1.vi" "电机上序状态"() -> (w356:refnum<vi>)
            n208 = global read "Global1.vi" "ECU上序状态"() -> (w358:refnum<vi>)
            n209 = case shown="\"追溯\"" w348 {
              tunnel: ["联网" ("connectionMode") "单机" ("connectionMode")] -> w361
              frame "追溯" {
              }
              frame "单机", Default {
              }
            }
            "connectionMode" <- w361
            n210 = call "Colour.vi"("result"="", "colourRef"=w356) -> ()  [unwired: 9 in, 1 out]
            n211 = global read "Global.vi" "管柱码"() -> (w351:refnum<vi>)
            n212 = call "Colour.vi"("result"="", "colourRef"=w358) -> ()  [unwired: 9 in, 1 out]
            n213 = global read "Global1.vi" "用户信息"() -> (w354:T6)
            n214 = Unbundle By Name(w354) -> ("用户名"=→"userName":string, "用户权限"=→"userStatus":string)
            n215 = global write "Global1.vi" "工位追溯码_ECU"(w350) -> ()
            n216 = property class="Str"(reference=w351, "Text.Text"=w350) -> ()  [unwired: 1 in, 2 out]
            n217 = global write "Global1.vi" "电机码"(w350) -> ()
            n218 = global write "Global1.vi" "控制器码"(w350) -> ()
            "安装支架数量" <- w359
            "产品型号" <- "" ("productsName")
            "电机安装数量" <- w359
          }
          frame #1 {
            n219 = control-ref of="更换产品"() -> (w371:refnum<vi>)
            n220 = control-ref of="电机自动"() -> (w373:refnum<vi>)
            n221 = control-ref of="ECU自动"() -> (w368:refnum<vi>)
            n222 = global write "Global.vi" "电机程序自动"(w373) -> ()
            n223 = global write "Global.vi" "ECU自动"(w368) -> ()
            n224 = control-ref of="批次信息"() -> (w375:refnum<vi>)
            n225 = control-ref of="ECU前序显示字"() -> (w366:refnum<vi>)
            n226 = control-ref of="上序状态"() -> (w365:refnum<vi>)
            n227 = global write "Global.vi" "更换产品"(w371) -> ()
            n228 = global write "Global.vi" "批次"(w375) -> ()
            n229 = control-ref of="模式切换"() -> (w364:refnum<vi>)
            n230 = global write "Global.vi" "ECU前序显示字"(w366) -> ()
            n231 = global write "Global.vi" "装配前序显示字"(w365) -> ()
            n232 = control-ref of="错误"() -> (w374:refnum<vi>)
            n233 = global write "Global.vi" "报警图标"(w374) -> ()
            n234 = global write "Global.vi" "模式切换"(w364) -> ()
            n235 = control-ref of="ECU结果显示"() -> (w367:refnum<vi>)
            n236 = control-ref of="提示信息"() -> (w372:refnum<vi>)
            n237 = control-ref of="安装支架数量"() -> (w370:refnum<vi>)
            n238 = control-ref of="检测结果"() -> (w369:refnum<vi>)
            n239 = global write "Global.vi" "提示信息"(w372) -> ()
            n240 = global write "Global.vi" "检测结果"(w369) -> ()
            n241 = global write "Global.vi" "安装支架生产数量"(w370) -> ()
            n242 = global write "Global.vi" "ECU结果显示"(w367) -> ()
          }
          frame #2 {
          }
          frame #3 {
            w387 = " " ("值")
            n243 = global read "Global.vi" "ECU结果显示"() -> (w393:refnum<vi>)
            n244 = vi-ref "A170316-11_config.vi"() -> (w396:refnum<vi>)
            n245 = control-ref of="ECU装配\n前序状态"() -> (w390:refnum<vi>)
            n246 = control-ref of="上序状态"() -> (w389:refnum<vi>)
            n247 = call "CallVI.vi"("VI引用"=w396, "状态"=T2."Standard") -> ()  [unwired: 11 in, 3 out]
            n248 = global write "Global1.vi" "ECU上序状态"(w390) -> ()
            n249 = global write "Global1.vi" "电机上序状态"(w389) -> ()
            n250 = property class="Str"(reference=w393, "Value"="..." ("结果显示")) -> (reference out=w392:refnum<vi>)  [unwired: 1 in, 1 out]
            n251 = vi-ref "A170316-11_Auto.vi"() -> (w380:refnum<vi>)
            n252 = global read "Global.vi" "装配前序显示字"() -> (w381:refnum<vi>)
            n253 = global read "Global.vi" "ECU前序显示字"() -> (w388:refnum<vi>)
            n254 = property class="Str"(reference=w392, "Text.TextColor"=u32 16776960) -> ()  [unwired: 1 in, 2 out]
            n255 = invoke class="VI" method="Ctrl Val.Set"(reference=w380, "Control Name"="STEP3" ("控件名"), "Value"="初始化" ("控件名")) -> ()  [unwired: 2 in, 5 out]
            n256 = call "看板状态.vi"("附加信息"="", "设备状态"=enum16{"设备离线", "设备正常", "设备缺料", "设备故障", "质量报警"}."设备正常") -> ("错误输出"=w385:errorcluster)  [unwired: 9 in]
            n257 = disable-structure shown="禁用" {
              frame Disabled {
                n258 = call "看板状态.vi"("附加信息"="", "设备状态"=enum16{"设备离线", "设备正常", "设备缺料", "设备故障", "质量报警"}."设备正常") -> ("错误输出"=w398:errorcluster)  [unwired: 9 in]
              }
              frame Enabled {
              }
            }
            n259 = property class="Str"(reference=w381, "Value"=w387) -> (reference out=w377:refnum<vi>)  [unwired: 1 in, 1 out]
            n260 = vi-ref "client.vi"() -> (w386:refnum<vi>)
            n261 = property class="Str"(reference=w388, "Value"=w387) -> ()  [unwired: 1 in, 2 out]
            n262 = property class="Str"(reference=w377, "Text.BGColor"=u32 16777216 ("文本.文本颜色:背景色")) -> ()  [unwired: 1 in, 2 out]
            n263 = call "CallVI.vi"("VI引用"=w386, "状态"=T2."Hidden", "错误输入"=w385) -> ()  [unwired: 10 in, 3 out]
            n264 = call "浮动通知.vi"("通知内容"="请选择产品") -> ()  [unwired: 11 in]
          }
        }
        n265 = call <vilib>:"Add State(s) to Queue__jki_lib_state_machine.vi"("State(s) in (\"\")"=w347) -> ("States Out"=w346:string)  [unwired: 14 in]
      }
      frame "UI: Cursor Set" {
        # "Argument"
        n266 = case shown="\"Busy\"" w402 {
          tunnel: w404 -> [w409 w411]
          tunnel: [w408 w410] -> w403
          frame "Idle", Default {
            n267 = call <vilib>:"Unset Busy.vi"("error in (no error)"=w409) -> ("error out"=w408:errorcluster)  [unwired: 10 in]
          }
          frame "Busy" {
            n268 = call <vilib>:"Set Busy.vi"("error in (no error)"=w411) -> ("error out"=w410:errorcluster)  [unwired: 9 in, 1 out]
          }
        }
        n269 = call <vilib>:"Add State(s) to Queue__jki_lib_state_machine.vi"("State(s) in (\"\")"=w407) -> ("States Out"=w406:string)  [unwired: 14 in]
      }
      frame "UI: Front Panel State" {
        # "Argument"
        n270 = Unbundle By Name(w415) -> ("Core.Current VI Reference"=w414:refnum<vi>)
        n271 = case shown="\"Open\", 默认" w413 {
          tunnel: w417 -> [w423 w436]
          tunnel: [w425 w437] -> w416
          tunnel: w414 -> [w424 w434]
          frame "Open", Default {
            n272 = property class="VI"(reference=w424, error in=w423) -> (reference out=w421:refnum<vi>, error out=w422:errorcluster, "Front Panel.Open"=w420:bool)
            n273 = case shown="假" w420 {
              tunnel: [w428 w431] -> w425
              tunnel: w422 -> [w427 w431]
              tunnel: w421 -> [w426 _]
              frame False {
                n274 = invoke class="VI" method="FP.Open"(reference=w426, error in=w427, "Activate"=TRUE, "State"=T2."Standard") -> (error out=w428:errorcluster)  [unwired: 1 in, 4 out]
              }
              frame True {
              }
            }
          }
          frame "Close" {
            n275 = property class="VI"(reference=w434, error in=w436) -> (reference out=w433:refnum<vi>, error out=w435:errorcluster, "Front Panel.Open"=w432:bool)
            n276 = case shown="真" w432 {
              tunnel: [w438 w441] -> w437
              tunnel: w435 -> [w438 w440]
              tunnel: w433 -> [_ w439]
              frame False {
              }
              frame True {
                n277 = invoke class="VI" method="FP.Close"(reference=w439, error in=w440) -> (error out=w441:errorcluster)  [unwired: 1 in, 2 out]
              }
            }
          }
        }
        n278 = call <vilib>:"Add State(s) to Queue__jki_lib_state_machine.vi"("State(s) in (\"\")"=w419) -> ("States Out"=w418:string)  [unwired: 14 in]
      }
      frame "---------- Macro ----------" {
        n279 = call <vilib>:"Add State(s) to Queue__jki_lib_state_machine.vi"("State(s) in (\"\")"=w446) -> ("States Out"=w445:string)  [unwired: 14 in]
      }
      frame "Macro: Initialize" {
        w448 = "Data: Initialize\nInitialize Core Data\nUI: Initialize\nUI: Init\nUI: Front Panel State >> Open"  # Data: Initialize Initialize Core Data UI: Initialize UI: Init UI: Front Panel State >> Open
        n280 = call <vilib>:"Add State(s) to Queue__jki_lib_state_machine.vi"("State(s) in Front (\"\")"=w448, "State(s) in (\"\")"=w452) -> ("States Out"=w451:string)  [unwired: 13 in]
      }
      frame "Macro: Exit" {
        n281 = Unbundle By Name(w465) -> ("Core.Close Panel on Exit?"=w464:bool)
        n282 = vi-ref "client.vi"() -> (w458:refnum<vi>)
        n283 = invoke class="VI" method="Abort VI"(reference=w458) -> (reference out=w457:refnum<vi>, error out=w456:errorcluster)  [unwired: 2 in, 1 out]
        n284 = invoke class="VI" method="FP.Close"(reference=w457, error in=w456) -> (reference out=w455:refnum<vi>, error out=w454:errorcluster)  [unwired: 1 in, 1 out]
        n285 = Select(t="UI: Front Panel State >> Close", s=w464, f="") -> (s? t:f=w461:string)
        n286 = Close Reference(reference=w455, error in (no error)=w454) -> ()  [unwired: 1 out]
        n287 = call <vilib>:"Add State(s) to Queue__jki_lib_state_machine.vi"("State(s) in (\"\")"=w461, "State(s) at Back (\"\")"="Data: Cleanup\nExit") -> ("States Out"=w459:string)  [unwired: 13 in]
        n288 = call <vilib>:"Add State(s) to Queue__jki_lib_state_machine.vi"("State(s) in Front (\"\")"=w459, "State(s) in (\"\")"=w468) -> ("States Out"=w467:string)  [unwired: 13 in]
      }
      frame "---------- New Category ----------" {
        n289 = call <vilib>:"Add State(s) to Queue__jki_lib_state_machine.vi"("State(s) in (\"\")"=w473) -> ("States Out"=w472:string)  [unwired: 14 in]
      }
      frame "New Category: 1" {
        n290 = call <vilib>:"Add State(s) to Queue__jki_lib_state_machine.vi"("State(s) in (\"\")"=w478) -> ("States Out"=w477:string)  [unwired: 14 in]
      }
      frame "New Category: 2" {
        n291 = call <vilib>:"Add State(s) to Queue__jki_lib_state_machine.vi"("State(s) in (\"\")"=w483) -> ("States Out"=w482:string)  [unwired: 14 in]
      }
    }
  }
  n292 = call-dynamic "Cleanup.vi"("MenuStrip in"=w1) -> ()  [unwired: 10 in, 1 out]
